vi "UHR-Fleezers Control (host) - 12.6.1.vi"() -> ()   [LabVIEW 2012] (continued)
        w3862 = u32 0 items=["Horizontal", "Vertical", "Central", "1st Diagonal", "2nd Diagonal"] ("Type of Symmetry")
        w3865 = u32 0 items=["Horizontal", "Vertical", "Central", "1st Diagonal", "2nd Diagonal"] ("Type of Symmetry")
        w3894 = u32 0 items=["Horizontal", "Vertical", "Central", "1st Diagonal", "2nd Diagonal"] ("Type of Symmetry")
        n2514 = Unbundle(w3802) -> (w3801:u32[], w3799:u32[], w3797:u32[])
        n2515 = To Double Precision Float(number=w3801) -> (double precision float=w3800:dbl[])
        n2516 = To Double Precision Float(number=w3799) -> (double precision float=w3798:dbl[])
        n2517 = To Double Precision Float(number=w3797) -> (double precision float=w3790:dbl[])
        n2518 = Index Array(array=w3923, index=10) -> (element=w3929:waveform(dbl))
        n2519 = Index Array(array=w3923, index=11) -> (element=w3926:waveform(dbl))
        n2520 = local read "Cycles/step (MCL)"() -> (w3879:u64)
        n2521 = Index Array(array=w3923, index="Channel") -> (element=w3925:waveform(dbl))
        n2522 = Unbundle(w3831) -> ("New Image"=w3830:T2, "New Image"=w3829:T2, "New Image"=w3803:T2, "New Image"=w3804:T2, "New Image"=w3805:T2)
        n2523 = local read "Scan steps (MCL)"() -> (w3792:u64)
        n2524 = Unbundle By Name(w3929) -> ("Y"=w3881:dbl[])
        n2525 = Unbundle By Name(w3926) -> ("Y"=w3883:dbl[])
        n2526 = local read "Scan lines (y)"() -> (w3793:u64)
        n2527 = local read "N APD Samp/step"() -> (w3795:dbl)
        n2528 = Unbundle By Name(w3925) -> ("Y"=w3888:dbl[])
        n2529 = call "downsample 1D array - double.vi"("Ave N"=w3879, "Array In"=w3881) -> ("Array Out"=w3880:dbl[])  [unwired: 1 out]
        n2530 = call "downsample 1D array - double.vi"("Ave N"=w3879, "Array In"=w3883) -> ("Array Out"=w3882:dbl[])  [unwired: 1 out]
        n2531 = call "downsample 1D array - double.vi"("Ave N"=w3879, "Array In"=w3888) -> ("Array Out"=w3887:dbl[])  [unwired: 1 out]
        n2532 = Multiply(x=w3792, y=u64 2) -> (x*y=w3794:u64)
        n2533 = feedback #11(w3798) -> (w3856:dbl[])
        n2534 = Build Array (concatenate)(w3856, w3798) -> (w3855:dbl[])
        n2535 = feedback #12(w3790) -> (w3791:dbl[])
        n2536 = Build Array (concatenate)(w3791, w3790) -> (w3789:dbl[])
        n2537 = Select(t=w3798, s=w3796, f=w3855) -> (s? t:f=w3840:dbl[])
        n2538 = feedback-in #11(w3840) -> ()
        n2539 = Select(t=w3790, s=w3796, f=w3789) -> (s? t:f=w3814:dbl[])
        n2540 = feedback-in #12(w3814) -> ()
        n2541 = feedback #13(w3800) -> (w3949:dbl[])
        n2542 = Build Array (concatenate)(w3949, w3800) -> (w3931:dbl[])
        n2543 = Select(t=w3800, s=w3796, f=w3931) -> (s? t:f=w3935:dbl[])
        n2544 = feedback-in #13(w3935) -> ()
        n2545 = feedback #14(w3880) -> (w3937:dbl[])
        n2546 = Build Array (concatenate)(w3937, w3880) -> (w3928:dbl[])
        n2547 = feedback #15(w3887) -> (w3947:dbl[])
        n2548 = Build Array (concatenate)(w3947, w3887) -> (w3946:dbl[])
        n2549 = feedback #16(w3882) -> (w3939:dbl[])
        n2550 = Build Array (concatenate)(w3939, w3882) -> (w3940:dbl[])
        n2551 = Select(t=w3880, s=w3796, f=w3928) -> (s? t:f=w3884:dbl[])
        n2552 = feedback-in #14(w3884) -> ()
        n2553 = Select(t=w3887, s=w3796, f=w3946) -> (s? t:f=w3886:dbl[])
        n2554 = feedback-in #15(w3886) -> ()
        n2555 = Select(t=w3882, s=w3796, f=w3940) -> (s? t:f=w3885:dbl[])
        n2556 = feedback-in #16(w3885) -> ()
        n2557 = call "integrate 1D array interval - double.vi"("Ave N"=w3795, "Array In"=w3840) -> ("Array Out"=w3851:dbl[])  [unwired: 1 out]
        n2558 = call "integrate 1D array interval - double.vi"("Ave N"=w3795, "Array In"=w3814) -> ("Array Out"=w3825:dbl[])  [unwired: 1 out]
        n2559 = call "integrate 1D array interval - double.vi"("Ave N"=w3795, "Array In"=w3935) -> ("Array Out"=w3934:dbl[])  [unwired: 1 out]
        n2560 = Array Size(array=w3851) -> (size(s)=w3852:i32)
        n2561 = Array Size(array=w3825) -> (size(s)=w3826:i32)
        n2562 = Array Size(array=w3934) -> (size(s)=w3936:i32)
        n2563 = Multiply(x=w3793, y=w3794) -> (x*y=w3854:u64)
        n2564 = Multiply(x=w3793, y=w3794) -> (x*y=w3828:u64)
        n2565 = Multiply(x=w3793, y=w3794) -> (x*y=w3944:u64)
        n2566 = Subtract(x=w3854, y=w3852) -> (x-y=w3845:u64)
        n2567 = call-poly <vilib>:"Mean.vi"("X"=w3851) -> ("mean"=w3842:dbl)  [unwired: 1 out]
        n2568 = Subtract(x=w3828, y=w3826) -> (x-y=w3819:u64)
        n2569 = call-poly <vilib>:"Mean.vi"("X"=w3825) -> ("mean"=w3816:dbl)  [unwired: 1 out]
        n2570 = Subtract(x=w3944, y=w3936) -> (x-y=w3878:u64)
        n2571 = call-poly <vilib>:"Mean.vi"("X"=w3934) -> ("mean"=w3875:dbl)  [unwired: 1 out]
        n2572 = call-poly <vilib>:"Mean.vi"("X"=w3884) -> ("mean"=w3868:dbl)  [unwired: 1 out]
        n2573 = call-poly <vilib>:"Mean.vi"("X"=w3886) -> ("mean"=w3873:dbl)  [unwired: 1 out]
        n2574 = call-poly <vilib>:"Mean.vi"("X"=w3885) -> ("mean"=w3871:dbl)  [unwired: 1 out]
        n2575 = Initialize Array(1.0 ("element"), w3845) -> (w3841:dbl[])
        n2576 = Initialize Array(1.0 ("element"), w3819) -> (w3815:dbl[])
        n2577 = Initialize Array(1.0 ("element"), w3878) -> (w3869:dbl[])
        n2578 = Multiply(x=w3841, y=w3842) -> (x*y=w3843:dbl[])
        n2579 = Multiply(x=w3815, y=w3816) -> (x*y=w3817:dbl[])
        n2580 = Multiply(x=w3869, y=w3875) -> (x*y=w3876:dbl[])
        n2581 = Multiply(x=w3869, y=w3871) -> (x*y=w3872:dbl[])
        n2582 = Multiply(x=w3869, y=w3873) -> (x*y=w3874:dbl[])
        n2583 = Multiply(x=w3869, y=w3868) -> (x*y=w3870:dbl[])
        n2584 = Build Array (concatenate)(w3851, w3843) -> (w3853:dbl[])
        n2585 = Build Array (concatenate)(w3825, w3817) -> (w3827:dbl[])
        n2586 = Build Array (concatenate)(w3934, w3876) -> (w3943:dbl[])
        n2587 = Build Array (concatenate)(w3884, w3870) -> (w3938:dbl[])
        n2588 = Build Array (concatenate)(w3886, w3874) -> (w3942:dbl[])
        n2589 = Build Array (concatenate)(w3885, w3872) -> (w3941:dbl[])
        n2590 = Reshape Array(w3853, w3793, w3794) -> (w3849:dbl[][])
        n2591 = Reshape Array(w3827, w3793, w3794) -> (w3823:dbl[][])
        n2592 = Reshape Array(w3943, w3793, w3794) -> (w3921:dbl[][])
        n2593 = Reshape Array(w3938, w3793, w3794) -> (w3904:dbl[][])
        n2594 = Reshape Array(w3942, w3793, w3794) -> (w3896:dbl[][])
        n2595 = Reshape Array(w3941, w3793, w3794) -> (w3911:dbl[][])
        n2596 = Array Subset(array=w3849, index (col)=0 ("index"), length (col)=w3792) -> (w3848:dbl[][])  [unwired: 2 in]
        n2597 = Array Subset(array=w3849, index (col)=w3792) -> (w3846:dbl[][])  [unwired: 3 in]
        n2598 = Array Subset(array=w3823, index (col)=0 ("index"), length (col)=w3792) -> (w3822:dbl[][])  [unwired: 2 in]
        n2599 = Array Subset(array=w3823, index (col)=w3792) -> (w3820:dbl[][])  [unwired: 3 in]
        n2600 = Array Subset(array=w3911, index (col)=0 ("index"), length (col)=w3792) -> (w3916:dbl[][])  [unwired: 2 in]
        n2601 = Array Subset(array=w3911, index (col)=w3792) -> (w3914:dbl[][])  [unwired: 3 in]
        n2602 = Array Subset(array=w3921, index (col)=0 ("index"), length (col)=w3792) -> (w3920:dbl[][])  [unwired: 2 in]
        n2603 = Array Subset(array=w3921, index (col)=w3792) -> (w3918:dbl[][])  [unwired: 3 in]
        n2604 = Array Subset(array=w3896, index (col)=0 ("index"), length (col)=w3792) -> (w3902:dbl[][])  [unwired: 2 in]
        n2605 = Array Subset(array=w3896, index (col)=w3792) -> (w3900:dbl[][])  [unwired: 3 in]
        n2606 = Array Subset(array=w3904, index (col)=0 ("index"), length (col)=w3792) -> (w3909:dbl[][])  [unwired: 2 in]
        n2607 = Array Subset(array=w3904, index (col)=w3792) -> (w3907:dbl[][])  [unwired: 3 in]
        n2608 = for {
          tunnel: w3848 -> [w3953] mode=indexing
          tunnel: [w3952] -> w3847 mode=indexing
          workers-P: _ -> [_]
          n2609 = Reverse 1D Array(array=w3953) -> (reversed array=w3952:dbl[])
        }
        n2610 = for {
          tunnel: w3822 -> [w3951] mode=indexing
          tunnel: [w3950] -> w3821 mode=indexing
          workers-P: _ -> [_]
          n2611 = Reverse 1D Array(array=w3951) -> (reversed array=w3950:dbl[])
        }
        n2612 = for {
          tunnel: w3916 -> [w3959] mode=indexing
          tunnel: [w3958] -> w3915 mode=indexing
          workers-P: _ -> [_]
          n2613 = Reverse 1D Array(array=w3959) -> (reversed array=w3958:dbl[])
        }
        n2614 = for {
          tunnel: w3920 -> [w3961] mode=indexing
          tunnel: [w3960] -> w3919 mode=indexing
          workers-P: _ -> [_]
          n2615 = Reverse 1D Array(array=w3961) -> (reversed array=w3960:dbl[])
        }
        n2616 = for {
          tunnel: w3902 -> [w3955] mode=indexing
          tunnel: [w3954] -> w3901 mode=indexing
          workers-P: _ -> [_]
          n2617 = Reverse 1D Array(array=w3955) -> (reversed array=w3954:dbl[])
        }
        n2618 = for {
          tunnel: w3909 -> [w3957] mode=indexing
          tunnel: [w3956] -> w3908 mode=indexing
          workers-P: _ -> [_]
          n2619 = Reverse 1D Array(array=w3957) -> (reversed array=w3956:dbl[])
        }
        n2620 = Index Array(array=w3921, index (row)=0) -> (element=→"Waveform Graph":dbl[])  [unwired: 1 in]
        n2621 = Add(x=w3847, y=w3846) -> (x+y=w3833:dbl[][])
        n2622 = Add(x=w3821, y=w3820) -> (x+y=w3807:dbl[][])
        n2623 = Add(x=w3915, y=w3914) -> (x+y=w3913:dbl[][])
        n2624 = Add(x=w3919, y=w3918) -> (x+y=w3893:dbl[][])
        n2625 = Add(x=w3901, y=w3900) -> (x+y=w3899:dbl[][])
        n2626 = Add(x=w3908, y=w3907) -> (x+y=w3906:dbl[][])
        n2627 = Divide(x=w3899, y=2) -> (x/y=w3897:dbl[][])
        n2628 = Divide(x=w3913, y=2) -> (x/y=w3858:dbl[][])
        n2629 = To Single Precision Float(number=w3893) -> (single precision float=w3892:sgl[][])
        n2630 = To Single Precision Float(number=w3833) -> (single precision float=w3837:sgl[][])
        n2631 = To Single Precision Float(number=w3807) -> (single precision float=w3811:sgl[][])
        n2632 = Divide(x=w3906, y=2) -> (x/y=w3860:dbl[][])
        n2633 = Transpose 2D Array(2D array=w3897) -> (transposed array=→"Data map":dbl[][])
        n2634 = To Single Precision Float(number=w3858) -> (single precision float=w3864:sgl[][])
        n2635 = To Single Precision Float(number=w3860) -> (single precision float=w3861:sgl[][])
        n2636 = call "IMAQ ArrayToImage"("Image Pixels (Float)"=w3892, "Image"=w3830) -> ("Image Out"=w3895:T2)  [unwired: 8 in, 1 out]
        n2637 = call "IMAQ ArrayToImage"("Image Pixels (Float)"=w3837, "Image"=w3829) -> ("Image Out"=w3839:T2)  [unwired: 8 in, 1 out]
        n2638 = call "IMAQ ArrayToImage"("Image Pixels (Float)"=w3811, "Image"=w3803) -> ("Image Out"=w3813:T2)  [unwired: 8 in, 1 out]
        n2639 = call "IMAQ ArrayToImage"("Image Pixels (Float)"=w3864, "Image"=w3804) -> ("Image Out"=w3866:T2)  [unwired: 8 in, 1 out]
        n2640 = call "IMAQ Symmetry"("Type of Symmetry"=w3894, "Image Src"=w3895) -> ("Image Dst Out"=w3890:T2)  [unwired: 3 in, 1 out]
        n2641 = call "IMAQ ArrayToImage"("Image Pixels (Float)"=w3861, "Image"=w3805) -> ("Image Out"=w3863:T2)  [unwired: 8 in, 1 out]
        n2642 = call "IMAQ Symmetry"("Type of Symmetry"=w3838, "Image Src"=w3839) -> ("Image Dst Out"=w3835:T2)  [unwired: 3 in, 1 out]
        n2643 = call "IMAQ Symmetry"("Type of Symmetry"=w3812, "Image Src"=w3813) -> ("Image Dst Out"=w3809:T2)  [unwired: 3 in, 1 out]
        n2644 = call "IMAQ Symmetry"("Type of Symmetry"=w3865, "Image Src"=w3866) -> ("Image Dst Out"=→"Detection Laser X":T2)  [unwired: 3 in, 1 out]
        n2645 = call "IMAQ Symmetry"("Type of Symmetry"=w3862, "Image Src"=w3863) -> ("Image Dst Out"=→"Detection Laser Y":T2)  [unwired: 3 in, 1 out]
        n2646 = call "IMAQ Set Simple Calibration"("Calibration Axis Info"=T36 {"Origin Pixel"={"X"=0.0, "Y"=0.0}, "Angle Relative to Horizontal (deg)"=0.0, "Axis Reference"=0}, "Grid Descriptor"=T37 {"X Step"=0.3, "Y Step"=0.3, "Unit"=enum."Undefined"}, "Image"=w3890) -> ("Calibrated Image"=→"APD 1":T2)  [unwired: 7 in, 1 out]
        n2647 = call "IMAQ Set Simple Calibration"("Calibration Axis Info"=T36 {"Origin Pixel"={"X"=0.0, "Y"=0.0}, "Angle Relative to Horizontal (deg)"=0.0, "Axis Reference"=0}, "Grid Descriptor"=T37 {"X Step"=0.3, "Y Step"=0.3, "Unit"=enum."Undefined"}, "Image"=w3835) -> ("Calibrated Image"=→"APD 2":T2)  [unwired: 7 in, 1 out]
        n2648 = call "IMAQ Set Simple Calibration"("Calibration Axis Info"=T36 {"Origin Pixel"={"X"=0.0, "Y"=0.0}, "Angle Relative to Horizontal (deg)"=0.0, "Axis Reference"=0}, "Grid Descriptor"=T37 {"X Step"=0.3, "Y Step"=0.3, "Unit"=enum."Undefined"}, "Image"=w3809) -> ("Calibrated Image"=→"APD 3":T2)  [unwired: 7 in, 1 out]
      }
    }
    n2649 = case "For computing FFTs for display" shown="True" "Compute FFT" {
      tunnel: w3306 -> [_ w4433]
      frame False {
      }
      frame True {
        n2650 = Build Array("FFT 1 Choice 1", "FFT 1 Choice 2", "FFT 2 Choice 1", "FFT 2 Choice 2") -> (w4426:u16[])
        n2651 = Array Size(array=w4433) -> (size(s)=w4432:i32)
        n2652 = feedback-in #17(w4426) -> ()
        n2653 = feedback #17(u16[] [100, 100, 100, 100]) -> (w4427:u16[])
        n2654 = feedback-in #18("# Spectra to Ave.") -> ()
        n2655 = feedback #18("# Spectra to Ave.") -> (w4424:dbl)
        n2656 = Not Equal?(x="# Spectra to Ave.", y=w4424) -> (x != y?=w4423:bool)
        n2657 = Not Equal?(x=w4426, y=w4427) -> (x != y?=w4425:bool)
        n2658 = feedback #19(1.0) -> (w4410:dbl)
        n2659 = Compound Arithmetic op=OR("Reset FFT", w4425, w4423) -> (w4408:bool)
        n2660 = Select(t=1.0, s=w4408, f=w4410) -> (s? t:f=w4412:dbl)
        n2661 = Greater?(x=w4412, y="# Spectra to Ave.") -> (0:w4431:bool)
        n2662 = Increment(x=w4412) -> (x+1=w4411:dbl)
        n2663 = feedback-in #19(w4411) -> ()
        n2664 = local read "DMA Update Period (s)"() -> (w4406:dbl)
        n2665 = Multiply(x="# Spectra to Ave.", y=w4406) -> (x*y=→"Ave. Time (s)":dbl)
        n2666 = Build Array(cluster{"f0":dbl, "df":dbl, "magnitude":dbl[]} {"f0"=0.0, "df"=0.0, "magnitude"=[]} ("PSD")) -> (w4415:cluster{"f0":dbl, "df":dbl, "magnitude":dbl[]}[])
        n2667 = Build Array(w4415, w4415, w4415, w4415) -> (w4417:T46)
        n2668 = feedback #20(w4417) -> (w4422:T46)
        n2669 = for {
          N: 4 -> [_]
          tunnel: w4426 -> [w4455] mode=indexing
          tunnel: w4433 -> [w4456]
          tunnel: w4432 -> [w4458]
          tunnel: w4408 -> [w4451]
          tunnel: w4431 -> [w4450]
          tunnel: "# Spectra to Ave." -> [w4449]
          tunnel: [w4448] -> w4421 mode=indexing
          tunnel: w4422 -> [w4453] mode=indexing
          tunnel: [w4452] -> w4409 mode=indexing
          tunnel: w4412 -> [w4447]
          n2670 = Less?(x=w4455, y=w4458) -> (x < y?=w4457:bool)
          n2671 = Index Array(array=w4456, index=w4455) -> (element=w4454:waveform(dbl))
          n2672 = case shown="True" w4457 {
            tunnel: w4454 -> [_ w4475]
            tunnel: w4453 -> [w4460 w4473]
            tunnel: [w4460 w4461] -> w4452
            tunnel: w4451 -> [_ w4472]
            tunnel: w4450 -> [_ w4465]
            tunnel: w4449 -> [_ w4464]
            tunnel: [cluster{"f0":dbl, "df":dbl, "magnitude":dbl[]} {"f0"=0.0, "df"=0.0, "magnitude"=[]} ("PSD") w4466] -> w4448
            tunnel: w4447 -> [_ w4463]
            frame False {
            }
            frame True {
              n2673 = call <vilib>:"Std Deviation and Variance.vi"("X"=w4475) -> ("mean"=w4476:dbl)  [unwired: 1 in, 2 out]
              n2674 = Subtract(x=w4475, y=w4476) -> (x-y=w4474:waveform(dbl))
              n2675 = xnode "Spectral Measurements"("Signals"=w4474) -> ("PSD"=w4468:cluster{"f0":dbl, "df":dbl, "magnitude":dbl[]})  [unwired: 1 in, 1 out]
              n2676 = case shown="False" w4472 {
                tunnel: w4473 -> [w4485 _]
                tunnel: [w4481 w4490] -> w4461
                tunnel: w4468 -> [w4484 w4491]
                tunnel: w4465 -> [w4483 _]
                frame False {
                  n2677 = Build Array (concatenate)(w4485, w4484) -> (w4482:cluster{"f0":dbl, "df":dbl, "magnitude":dbl[]}[])
                  n2678 = case shown="True" w4483 {
                    tunnel: w4482 -> [w4486 w4489]
                    tunnel: [w4486 w4487] -> w4481
                    frame False {
                    }
                    frame True {
                      n2679 = Delete From Array(array=w4489, index=0) -> (array with subset deleted=w4487:cluster{"f0":dbl, "df":dbl, "magnitude":dbl[]}[])  [unwired: 1 in, 1 out]
                    }
                  }
                }
                frame True {
                  n2680 = Build Array(w4491) -> (w4490:cluster{"f0":dbl, "df":dbl, "magnitude":dbl[]}[])
                }
              }
              n2681 = for {
                tunnel: w4461 -> [w4480] mode=indexing
                tunnel: [w4479] -> w4471 mode=indexing
                workers-P: _ -> [_]
                n2682 = Unbundle By Name(w4480) -> ("magnitude"=w4479:dbl[])
              }
              n2683 = Transpose 2D Array(2D array=w4471) -> (transposed array=w4470:dbl[][])
              n2684 = for {
                tunnel: w4470 -> [w4478] mode=indexing
                tunnel: [w4477] -> w4469 mode=indexing
                workers-P: _ -> [_]
                n2685 = Add Array Elements(numeric array=w4478) -> (sum=w4477:dbl)
              }
              n2686 = Select(t=w4464, s=w4465, f=w4463) -> (s? t:f=w4462:dbl)
              n2687 = Divide(x=w4469, y=w4462) -> (x/y=w4467:dbl[])
              n2688 = Bundle By Name(cluster=w4468, "magnitude"=w4467) -> (w4466:cluster{"f0":dbl, "df":dbl, "magnitude":dbl[]})
            }
          }
        }
        n2689 = case shown="True" w4408 {
          tunnel: w4409 -> [w4440 w4446]
          tunnel: [w4440 w4441] -> w4407
          frame False {
          }
          frame True {
            n2690 = Array Subset(array=w4446, index (row)=0 ("index"), length (row)=4 ("length"), index (col)=0 ("index"), length (col)=1 ("length")) -> (w4441:T46)
          }
        }
        n2691 = feedback-in #20(w4407) -> ()
        n2692 = Split 1D Array(array=w4421, index=2) -> (first subarray=→"FFT 1":cluster{"f0":dbl, "df":dbl, "magnitude":dbl[]}[], second subarray=→"FFT 2":cluster{"f0":dbl, "df":dbl, "magnitude":dbl[]}[])
      }
    }
    n2693 = Index Array(array=w3304, index=4) -> (element=w3360:waveform(dbl))
    n2694 = Index Array(array=w3304, index=7) -> (element=w3357:waveform(dbl))
    n2695 = Divide(x="T1 offset_x (mV)", y=1000.0) -> (x/y=w3361:dbl)
    n2696 = feedback-in #21("Calibration") -> ()
    n2697 = feedback #21(u16 1 ("Calibration")) -> (w3379:u16)
    n2698 = Divide(x="T2 offset_x (mV)", y=1000.0) -> (x/y=w3359:dbl)
    n2699 = case shown="2" "Calibration" {
      tunnel: "T1 alpha_x (nm/V)" -> [_ w3754 w3775]
      tunnel: "T1 kappa_x (pN/nm)" -> [_ _ w3765]
      tunnel: "T2 alpha_x (nm/V)" -> [_ w3753 w3773]
      tunnel: "T2 kappa_x (pN/nm)" -> [_ _ w3766]
      tunnel: w3360 -> [w3736 w3751 w3771]
      tunnel: w3357 -> [w3735 w3749 w3769]
      tunnel: [w3736 w3748 w3768] -> w3388
      tunnel: [w3735 w3747 w3767] -> w3387
      tunnel: ["T1 X (V)" ("Label.Text") "T1 X (nm)" ("Label.Text") "T1 X (pN)" ("Label.Text")] -> w3376
      tunnel: ["T2 X (V)" ("Label.Text") "T2 X (nm)" ("Label.Text") "T2 X (pN)" ("Label.Text")] -> w3375
      tunnel: ["Position (V)" ("Label.Text") "Position (nm)" ("Label.Text") "Force (pN)" ("Label.Text")] -> w3377
      tunnel: w3359 -> [_ w3739 w3758]
      tunnel: w3361 -> [_ w3742 w3760]
      tunnel: ["Mean (V)" ("Label.Text") "Mean (nm)" ("Label.Text") "Mean (pN)" ("Label.Text")] -> w3372
      tunnel: ["Difference (V)" ("Label.Text") "Difference (nm)" ("Label.Text") "Difference (pN)" ("Label.Text")] -> w3312
      frame 0, Default {
      }
      frame 1 {
        n2700 = Unbundle By Name(w3751) -> ("Y"=w3755:dbl[])
        n2701 = Unbundle By Name(w3749) -> ("Y"=w3740:dbl[])
        n2702 = Subtract(x=w3755, y=w3742) -> (x-y=w3743:dbl[])
        n2703 = Subtract(x=w3740, y=w3739) -> (x-y=w3741:dbl[])
        n2704 = Multiply(x=w3741, y=w3753) -> (x*y=w3750:dbl[])
        n2705 = Multiply(x=w3754, y=w3743) -> (x*y=w3752:dbl[])
        n2706 = Bundle By Name(cluster=w3749, "Y"=w3750) -> (w3747:waveform(dbl))
        n2707 = Bundle By Name(cluster=w3751, "Y"=w3752) -> (w3748:waveform(dbl))
      }
      frame 2 {
        n2708 = Unbundle By Name(w3771) -> ("Y"=w3776:dbl[])
        n2709 = Unbundle By Name(w3769) -> ("Y"=w3774:dbl[])
        n2710 = Subtract(x=w3774, y=w3758) -> (x-y=w3759:dbl[])
        n2711 = Subtract(x=w3776, y=w3760) -> (x-y=w3761:dbl[])
        n2712 = Compound Arithmetic op=MULTIPLY(w3759, w3773, w3766) -> (w3770:dbl[])
        n2713 = Compound Arithmetic op=MULTIPLY(w3765, w3775, w3761) -> (w3772:dbl[])
        n2714 = Bundle By Name(cluster=w3769, "Y"=w3770) -> (w3767:waveform(dbl))
        n2715 = Bundle By Name(cluster=w3771, "Y"=w3772) -> (w3768:waveform(dbl))
      }
    }
    n2716 = case shown="True" "Read Lateness and Rel Phase" {
      tunnel: w3178 -> [w3690 w3724]
      tunnel: w3177 -> [w3691 w3723]
      tunnel: [w3690 w3696] -> w3354
      tunnel: [w3691 w3695] -> w3353
      frame False {
      }
      frame True {
        n2717 = xnode "Read/Write Control"("FPGA VI Reference In"=w3724, "error in"=w3723) -> ("FPGA VI Reference Out"=w3698:T20, "error out"=w3697:errorcluster, "GI Relative phase"=→"GI relative phase":i16, "Relative phase"=→"Relative phase (AI1)":i16, "AI Late Counter"=→"Late Counter (AI1)":u8, "GI Late Counter"=→"GI Late Counter":u8, "MCL Late Counter"=→"MCL Late Counter":u8, "MCL Relative Phase"=→"Relative Phase (MCL)":i16, "APD Acq Relative Phase"=→"APD Acq Relative Phase":i16, "APD 1 Gate Relative Phase"=→"APD 1 Gate Relative Phase":i16, "APD 2 Gate Relative Phase"=→"APD 2 Gate Relative Phase":i16, "APD Acq Late Counter"=→"APD Acq Late Counter":u8, "APD 1 Gate Late Counter"=→"APD 1 Gate Late Counter":u8, "APD 2 Gate Late Counter"=→"APD 2 Gate Late Counter":u8, "Green FB Relative Phase"=→"Relative phase (Green FB)":i16, "GI Relative phase 2"=→"GI relative phase 2":i16, "GI Late Counter 2"=→"GI Late Counter 2":u8, "Trap Pos FIFO Timeout"=→"Trap Pos FIFO Timeout":u16, "Trap AI FIFO Timeout"=→"Trap AI FIFO Timeout":u16, "RI Late Counter"=→"RI Late Counter":u8, "RI Relative phase"=→"RI relative phase":i16, "Green Late Counter"=→"Green AI Late Counter":u8, "BI Late Counter (AO)"=→"Late Counter (BI AO)":u8, "Blue Late Counter (D)"=→"Late Counter (BI DO)":u8, "BI Relative phase (AO)"=→"Relative phase (BI AO)":i16, "BI Relative phase (D)"=→"Relative phase (BI DO)":i16, "DIO Relative phase"=→"DIO Relative phase":i16)
        n2718 = xnode "Read/Write Control"("FPGA VI Reference In"=w3698, "error in"=w3697) -> ("FPGA VI Reference Out"=w3696:T20, "error out"=w3695:errorcluster, "APD 3 Gate Late Counter"=→"APD 3 Gate Late Counter":u8, "APD 3 Gate Relative Phase"=→"APD 3 Gate Relative Phase":i16)
      }
    }
    n2719 = Not Equal?(x=w3379, y="Calibration") -> (x != y?=w3338:bool)
    n2720 = case shown="True" w3338 {
      tunnel: w3377 -> [_ w3729]
      tunnel: w3376 -> [_ w3728]
      tunnel: w3375 -> [_ w3727]
      tunnel: w3372 -> [_ w3726]
      tunnel: w3312 -> [_ w3725]
      frame False {
      }
      frame True {
        n2721 = property on="Force" class="WFChart (strict)"("YScale.NameLbl.Text"=w3729) -> ()  [unwired: 2 in, 2 out]
        n2722 = property on="T2 X" class="DigNum (strict)"("Caption.Text"=w3727) -> ()  [unwired: 2 in, 2 out]
        n2723 = property on="T1 X" class="DigNum (strict)"("Caption.Text"=w3728) -> ()  [unwired: 2 in, 2 out]
        n2724 = property on="Mean" class="DigNum (strict)"("Caption.Text"=w3726) -> ()  [unwired: 2 in, 2 out]
        n2725 = property on="Difference" class="DigNum (strict)"("Caption.Text"=w3725) -> ()  [unwired: 2 in, 2 out]
      }
    }
    n2726 = Unbundle By Name(w3360) -> ("Y"=w3363:dbl[])
    n2727 = Unbundle By Name(w3357) -> ("Y"=w3366:dbl[])
    n2728 = Subtract(x=w3363, y=w3361) -> (x-y=w3364:dbl[])
    n2729 = Subtract(x=w3366, y=w3359) -> (x-y=w3365:dbl[])
    n2730 = Multiply(x=w3365, y="T2 alpha_x (nm/V)") -> (x*y=w3160:dbl[])
    n2731 = Multiply(x="T1 alpha_x (nm/V)", y=w3364) -> (x*y=w3161:dbl[])
    n2732 = Not(x="Trap Trig. Fl.") -> (.not. x?=w3197:bool)
    n2733 = Multiply(x=w3387, y=-1.0) -> (x*y=w3368:waveform(dbl))
    n2734 = Subtract(x=w3161, y=w3160) -> (x-y=w3356:dbl[])
    n2735 = Unbundle By Name(w3387) -> ("Y"=w3328:dbl[])
    n2736 = Unbundle By Name(w3388) -> ("Y"=w3162:dbl[])
    n2737 = Negate(x=w3356) -> (-x=w3158:dbl[])
    n2738 = Build Array(w3388, w3368) -> (→"Force":waveform(dbl)[])
    n2739 = Subtract(x=w3158, y="Offset (nm)") -> (x-y=w3326:dbl[])
    n2740 = call-poly <vilib>:"Mean.vi"("X"=w3328) -> ("mean"=w3164:dbl)  [unwired: 1 out]
    "T2 X" <- w3164
    n2741 = Negate(x=w3328) -> (-x=w3329:dbl[])
    n2742 = call-poly <vilib>:"Mean.vi"("X"=w3162) -> ("mean"=w3165:dbl)  [unwired: 1 out]
    "T1 X" <- w3165
    n2743 = Negate(x=w3164) -> (-x=w3163:dbl)
    n2744 = Bundle By Name(cluster=w3360, "Y"=w3326) -> (w3303:waveform(dbl))
    "Bead Separation" <- w3303
    n2745 = Add(x=w3162, y=w3329) -> (x+y=w3330:dbl[])
    n2746 = Add(x=w3165, y=w3163) -> (x+y=w3374:dbl)
    n2747 = Subtract(x=w3165, y=w3163) -> (x-y=→"Difference":dbl)
    n2748 = Divide(x=w3330, y=2.0) -> (x/y=→"Vec Mean of T1 T2":dbl[])
    n2749 = Divide(x=w3374, y=2.0) -> (x/y=w3332:dbl)
    "Mean" <- w3332
    n2750 = feedback-in #22("Trap Trig. Fl.") -> ()
    n2751 = feedback #22("Trap Trig. Fl.") -> (w3195:bool)
    n2752 = And(x=w3197, y=w3195) -> (x .and. y?=w3196:bool)
    n2753 = case "If have just turned off triggering" shown="True" w3196 {
      tunnel: w3178 -> [_ w3525]
      tunnel: w3177 -> [_ w3524]
      frame False {
      }
      frame True {
        w3523 = FALSE ("FPGA Trap Trig")
        n2754 = xnode "Read/Write Control"("FPGA VI Reference In"=w3525, "error in"=w3524, "FPGA Trap Trig"=w3523) -> ("FPGA VI Reference Out"=w3522:T20, "error out"=w3521:errorcluster)
        n2755 = xnode "Read/Write Control"("FPGA VI Reference In"=w3522, "error in"=w3521, "TTrig?"=w3523) -> ()  [unwired: 2 out]
        n2756 = local write "Initializing"(FALSE ("Initializing")) -> ()
        n2757 = local write "Triggered"(FALSE ("Triggered")) -> ()
        n2758 = local write "Waiting"(FALSE ("Waiting")) -> ()
      }
    }
    n2759 = Not(x=w3195) -> (.not. x?=w3208:bool)
    n2760 = And(x="Trap Trig. Fl.", y=w3208) -> (x .and. y?=w3205:bool)
    n2761 = local read "Tether"() -> (w3333:bool)
    n2762 = Or(x=w3205, y="Reinitialize") -> (x .or. y?=w3191:bool)
    n2763 = feedback #23(w3201) -> (w3206:string)
    n2764 = Select(t=w3201, s=w3205, f=w3206) -> (s? t:f=w3200:string)
    n2765 = Select(t=w3201, s="Reinitialize", f=w3200) -> (s? t:f=w3199:string)
    n2766 = feedback #24(0) -> (w3203:i32)
    n2767 = feedback #25(w3326) -> (w3325:dbl[])
    n2768 = Build Array (concatenate)(w3326, w3325) -> (w3159:dbl[])
    n2769 = case "For determining if there is a tether still" shown="True" w3333 {
      tunnel: w3332 -> [_ w3649]
      frame False {
      }
      frame True {
        n2770 = Greater?(x="Lost Tether Alarm Threshold (pN)", y=w3649) -> (0:w3647:bool)
        n2771 = case shown="True" w3647 {
          frame False {
          }
          frame True {
            w3650 = FALSE ("Value (Signaling)")
            n2772 = flat-sequence {
              frame #0 {
                # "stop only if saving"
                n2773 = local read "Saving..."() -> (w3662:bool)
                n2774 = And(x=w3662, y="TA Cancel Save?") -> (x .and. y?=w3661:bool)
                n2775 = local write "Stop Saving"(w3661) -> ()
              }
              frame #1 {
                n2776 = case shown="True" "TA Green Off?" {
                  frame False {
                  }
                  frame True {
                    w3665 = FALSE ("Fl. Triggered...")
                    n2777 = local write "Fl. Triggered..."(w3665) -> ()
                    n2778 = property on="Green Laser ON" class="Bool (strict)"("Val(Sgnl)"=w3665) -> ()  [unwired: 2 in, 2 out]
                  }
                }
              }
            }
            n2779 = local read "Time tether formed"() -> (w3656:timestamp)
            n2780 = Get Date/Time In Seconds() -> (seconds since 1Jan1904=w3657:timestamp)
            n2781 = Subtract(x=w3657, y=w3656) -> (x-y=w3655:dbl)
            n2782 = Number To Decimal String(number=w3655) -> (decimal integer string=w3652:string)  [unwired: 1 out]
            n2783 = local read "Messages"() -> (w3659:string)
            n2784 = call <vilib>:"Beep.vi"() -> ()  [unwired: 3 in, 9 out]
            n2785 = Concatenate Strings("Lost tether (" ("Message to add"), w3652, " s)." ("string")) -> (w3654:string)
            n2786 = local write "Tether"(FALSE ("Tether")) -> ()
            n2787 = call "Update messages.vi"("Message to add"=w3654, "Old message string"=w3659) -> ("New message string"=w3658:string)
            n2788 = local write "Messages"(w3658) -> ()
            n2789 = property on="Fl. Triggered..." class="Bool (strict)"("Val(Sgnl)"=w3650) -> ()  [unwired: 2 in, 2 out]
            n2790 = local write "Dip for Protein"(w3650) -> ()
            n2791 = property on="Trap Pos. FB ON" class="Bool (strict)"("Val(Sgnl)"=w3650) -> ()  [unwired: 2 in, 2 out]
            n2792 = property on="Trap Trig. Fl." class="Bool (strict)"("Val(Sgnl)"=w3650) -> ()  [unwired: 2 in, 2 out]
          }
        }
      }
    }
    n2793 = case "For triggering actions based on the trap position (e.g., turning the excitation laser on if trap under feedback moves so far)" shown="True" "Trap Trig. Fl." {
      tunnel: w3186 -> [_ w3538]
      tunnel: w3199 -> [_ w3537]
      tunnel: ["" ("t") w3536] -> w3207
      tunnel: w3191 -> [_ w3535]
      tunnel: [0 ("t") w3534] -> w3204
      tunnel: w3203 -> [_ w3533]
      tunnel: w3178 -> [_ w3532]
      tunnel: w3177 -> [_ w3531]
      frame False {
      }
      frame True {
        n2794 = case shown="\"Wait for trigger\"" w3537 {
          tunnel: w3538 -> [w3555 _ _ w3603]
          tunnel: [w3552 w3584 "" ("t") w3606] -> w3536
          tunnel: w3535 -> [_ _ _ w3594]
          tunnel: [w3551 w3581 0 ("t") w3595] -> w3534
          tunnel: w3533 -> [_ w3583 _ w3601]
          tunnel: w3532 -> [w3540 w3578 _ w3597]
          tunnel: w3531 -> [w3539 w3577 _ w3596]
          frame "Wait for trigger" {
            n2795 = local read "Trap Trig. (FPGA)"() -> (w3543:bool)
            n2796 = Subtract(x=w3555, y="Mean T1 Position\nto compare (nm)") -> (x-y=w3548:dbl[])
            n2797 = call <vilib>:"Std Deviation and Variance.vi"("X"=w3548) -> ("mean"=→"mean":dbl, "standard deviation"=→"standard\ndeviation":dbl)  [unwired: 1 in, 1 out]
            n2798 = Array Max & Min(array=w3548) -> (max value=→"max value":dbl, min value=→"min value":dbl)  [unwired: 2 out]
            n2799 = Greater?(x=w3548, y="Threshold (nm)") -> (0:w3558:bool[])
            n2800 = case shown="True" w3543 {
              tunnel: w3540 -> [_ w3564]
              tunnel: w3539 -> [_ w3563]
              tunnel: [FALSE ("TTrig?") w3562] -> w3546
              frame False {
              }
              frame True {
                n2801 = xnode "Read/Write Control"("FPGA VI Reference In"=w3564, "error in"=w3563) -> ("TTrig?"=w3562:bool)  [unwired: 2 out]
              }
            }
            n2802 = Or Array Elements(Boolean array=w3558) -> (logical OR=w3545:bool)
            n2803 = Select(t=w3546, s=w3543, f=w3545) -> (s? t:f=w3544:bool)
            n2804 = Not(x=w3543) -> (.not. x?=w3542:bool)
            n2805 = And(x=w3544, y=w3542) -> (x .and. y?=w3541:bool)
            n2806 = Select(t="Triggered", s=w3544, f="Wait for trigger") -> (s? t:f=w3552:string)
            n2807 = case shown="True" w3544 {
              tunnel: [0 0] -> w3551
              tunnel: w3540 -> [_ w3569]
              tunnel: w3539 -> [_ w3568]
              frame False {
                "Waiting" <- TRUE ("Waiting")
              }
              frame True {
                n2808 = xnode "Read/Write Control"("FPGA VI Reference In"=w3569, "error in"=w3568, "TTrig?"=FALSE) -> ()  [unwired: 2 out]
                n2809 = local read "Messages"() -> (w3572:string)
                n2810 = call <vilib>:"Beep.vi"() -> ()  [unwired: 12 in]
                n2811 = call "Update messages.vi"("Message to add"="Unwinding trigger.", "Old message string"=w3572) -> ("New message string"=w3573:string)
                n2812 = local write "Messages"(w3573) -> ()
                n2813 = local write "Waiting"(FALSE ("Waiting")) -> ()
                "Triggered" <- TRUE ("Triggered")
              }
            }
            n2814 = case "Only need to turn on laser if host triggered" shown="True" w3541 {
              frame False {
              }
              frame True {
                n2815 = property on="Green Laser ON" class="Bool (strict)"("Val(Sgnl)"=TRUE ("Value (Signaling)")) -> ()  [unwired: 2 in, 2 out]
              }
            }
          }
          frame "Triggered" {
            n2816 = local read "Trap Trig. (FPGA)"() -> (w3580:bool)
            n2817 = Increment(x=w3583) -> (x+1=w3581:i32)
            n2818 = Greater Or Equal?(x=w3581, y="Fl. ON time (n)") -> (x >= y?=w3579:bool)
            n2819 = Select(t="Wait for trigger", s=w3579, f="Triggered" ("t")) -> (s? t:f=w3584:string)
            n2820 = And(x=w3579, y=w3580) -> (x .and. y?=w3576:bool)
            n2821 = case shown="True" w3576 {
              tunnel: w3578 -> [_ w3588]
              tunnel: w3577 -> [_ w3587]
              frame False {
              }
              frame True {
                n2822 = xnode "Read/Write Control"("FPGA VI Reference In"=w3588, "error in"=w3587, "FPGA Trap Trig"=TRUE) -> ()  [unwired: 2 out]
              }
            }
            n2823 = case shown="True" w3579 {
              frame False {
              }
              frame True {
                w3590 = FALSE ("Value (Signaling)")
                n2824 = local write "Triggered"(w3590) -> ()
                n2825 = local write "Waiting"(TRUE ("Waiting")) -> ()
                n2826 = property on="Green Laser ON" class="Bool (strict)"("Val(Sgnl)"=w3590) -> ()  [unwired: 2 in, 2 out]
              }
            }
          }
          frame "Do nothing" {
          }
          frame "Initialize", Default {
            n2827 = Increment(x=w3601) -> (x+1=w3605:i32)
            n2828 = Select(t=1, s=w3594, f=w3605) -> (s? t:f=w3595:i32)
            n2829 = feedback #26(w3603) -> (w3609:dbl[])
            n2830 = Build Array (concatenate)(w3603, w3609) -> (w3602:dbl[])
            n2831 = Greater Or Equal?(x=w3595, y="Wait to get offset (n)") -> (x >= y?=w3598:bool)
            n2832 = Select(t=w3603, s=w3594, f=w3602) -> (s? t:f=w3604:dbl[])
            n2833 = feedback-in #26(w3604) -> ()
            n2834 = call-poly <vilib>:"Mean.vi"("X"=w3604) -> ("mean"=w3599:dbl)  [unwired: 1 out]
            n2835 = local write "Mean T1 Position\nto compare (nm)"(w3599) -> ()
            n2836 = case shown="True" w3594 {
              tunnel: w3597 -> [_ w3615]
              tunnel: w3596 -> [_ w3614]
              frame False {
              }
              frame True {
                w3611 = FALSE ("FPGA Trap Trig")
                n2837 = xnode "Read/Write Control"("FPGA VI Reference In"=w3615, "error in"=w3614, "FPGA Trap Trig"=w3611) -> ("FPGA VI Reference Out"=w3613:T20, "error out"=w3612:errorcluster)
                n2838 = xnode "Read/Write Control"("FPGA VI Reference In"=w3613, "error in"=w3612, "TTrig?"=w3611) -> ()  [unwired: 2 out]
              }
            }
            n2839 = Select(t="Wait for trigger", s=w3598, f="Initialize") -> (s? t:f=w3606:string)
            n2840 = case shown="True" w3598 {
              tunnel: w3599 -> [_ w3618]
              tunnel: w3597 -> [_ w3627]
              tunnel: w3596 -> [_ w3626]
              frame False {
                n2841 = local write "Waiting"(FALSE ("Waiting")) -> ()
                "Initializing" <- TRUE ("Initializing")
              }
              frame True {
                n2842 = local read "Threshold (nm)"() -> (w3630:dbl)
                n2843 = local read "AOM X Cal (nm/MHz)"() -> (w3629:dbl)
                n2844 = Add(x=w3618, y=w3630) -> (x+y=w3631:dbl)
                n2845 = Divide(x=w3631, y=w3629) -> (x/y=w3628:dbl)
                n2846 = call "IR AOM freq to word.vi"("Frequency In (MHz)"=w3628) -> ("Frequency Word Out (double)"=w3625:dbl)
                n2847 = local write "Initializing"(FALSE ("Initializing")) -> ()
                n2848 = local write "Waiting"(TRUE ("Waiting")) -> ()
                n2849 = To Quad Integer(1:w3625) -> (0:w3624:i64)
                n2850 = xnode "Read/Write Control"("FPGA VI Reference In"=w3627, "error in"=w3626, "FPGA TTrig Thresh"=w3624) -> ("FPGA VI Reference Out"=w3621:T20, "error out"=w3620:errorcluster)
                n2851 = xnode "Read/Write Control"("FPGA VI Reference In"=w3621, "error in"=w3620, "FPGA Trap Trig"=TRUE) -> ()  [unwired: 2 out]
              }
            }
          }
        }
      }
    }
    n2852 = feedback-in #23(w3207) -> ()
    n2853 = feedback-in #24(w3204) -> ()
    n2854 = Split 1D Array(array=w3159, index=w3221) -> (first subarray=w3322:dbl[])  [unwired: 1 out]
    n2855 = feedback-in #25(w3322) -> ()
    n2856 = call-poly <vilib>:"Mean.vi"("X"=w3322) -> ("mean"=w3321:dbl)  [unwired: 1 out]
    "Bead Mean (nm)" <- w3321
    n2857 = Subtract(x=w3322, y=w3321) -> (x-y=w3320:dbl[])
    n2858 = Square(x=w3320) -> (x^2=w3319:dbl[])
    n2859 = call-poly <vilib>:"Mean.vi"("X"=w3319) -> ("mean"=w3318:dbl)  [unwired: 1 out]
    n2860 = Square Root(x=w3318) -> (sqrt(x)=w3317:dbl)
    n2861 = Multiply(x=10.0, y=w3317) -> (x*y=→"RMS (Ang)":dbl)
    n2862 = xnode ("Read/Write Control")("FPGA VI Reference In"=w3354, "error in"=w3353) -> ("FPGA VI Reference Out"=w3189:T20, "error out"=w3188:errorcluster, "AI2 Y Sum Set 1"=w3452:i16, "AI2 Y Sum Set 2"=w3451:i16, "AI1 X Set 1"=w3253:fxp<+/-,16,1>, "AI1 X Set 2"=w3252:fxp<+/-,16,1>, "Trap Pos FB Int Signal"=→"Trap Pos FB Int Signal":fxp<+/-,24,9>, "Trap Pos FB Int-Norm Signal"=→"Trap Pos FB Int-Norm Signal":fxp<+/-,16,1>, "Trap Pos FB Action"=w3246:i64, "Scanning"=→"AOD Scanning":bool, "Scan I"=→"AOD Scan I":u64, "Scanning MCL"=w3454:bool, "Scan I (MCL)"=→"MCL Scan I":u64, "Green FB Sum"=w3391:i16, "Trap Pos FB Action"=w3176:i64, "TTrig Fin Thresh"=w3172:i64, "Red FB Intensity"=w3153:i16, "Blue Intensity"=w3148:i16)
    "MCL Scanning" <- w3454
    "Trap Pos FB Action" <- w3246
    n2863 = Divide(x=w3153, y=3276.7) -> (x/y=w3152:dbl)
    "Red laser intensity (V)" <- w3152
    n2864 = Divide(x=w3148, y=3276.7) -> (x/y=w3147:dbl)
    "Blue laser intensity (V)" <- w3147
    n2865 = Divide(x=w3391, y=3276.7) -> (x/y=w3151:dbl)
    "Green laser intensity (V)" <- w3151
    n2866 = local read "FB Trig Integrate"() -> (w3170:u32)
    n2867 = Divide(x=w3176, y=w3170) -> (x/y=w3169:dbl)
    "TTrig Sig (Int)" <- w3169
    n2868 = Bundle(w3151, w3152, w3147) -> (→"Fluorescence laser intensities plot":cluster{dbl, dbl, dbl})  [unwired: 1 in]
    n2869 = Divide(x=w3172, y=w3170) -> (x/y=w3167:dbl)
    "TTrig Fin Thresh (Int)" <- w3167
    n2870 = local read "AOM X Cal (nm/MHz)"() -> (w3175:dbl)
    n2871 = local read "AI2 (V)"() -> (w3453:cluster{"Set 1":dbl, "Set 2":dbl})
    n2872 = Bundle By Name(cluster=w3453, "Set 1"=w3452, "Set 2"=w3451) -> (w3449:cluster{"Set 1":dbl, "Set 2":dbl})
    n2873 = Divide(x=w3246, y=327.67) -> (x/y=→"Action (%)":dbl)
    n2874 = local read "Trap X (AI1)"() -> (w3266:T10)
    n2875 = call "IR AOM word double to freq.vi"("Frequency Word In (double)"=w3167) -> ("Frequency Out (MHz)"=w3166:dbl)
    n2876 = call "IR AOM word double to freq.vi"("Frequency Word In (double)"=w3169) -> ("Frequency Out (MHz)"=w3168:dbl)
    n2877 = Divide(x=w3449, y=3276.7) -> (x/y=w3448:cluster{"Set 1":dbl, "Set 2":dbl})
    n2878 = Multiply(x=w3168, y=w3175) -> (x*y=w3174:dbl)
    "TTrig Sig (nm)" <- w3174
    n2879 = Multiply(x=w3166, y=w3175) -> (x*y=w3173:dbl)
    "TTrig Fin Thresh (nm)" <- w3173
    n2880 = local write "AI2 (V)"(w3448) -> ()
    n2881 = Bundle(cluster=w3266, "Trap 1"=w3253, "Trap 2"=w3252) -> (→"Trap X (AI1)":T10)
    n2882 = Bundle(w3174, w3173) -> (→"TTrig":cluster{dbl, dbl})  [unwired: 1 in]
    n2883 = flat-sequence "To save data" {
      tunnel: [w4539] -> w3472
      tunnel: [w4540] -> w3471
      tunnel: w3422 -> [w4533]
      tunnel: w3194 -> [w4537]
      tunnel: ["Save Calibration"] -> w3445
      tunnel: w3442 -> [w4536]
      tunnel: [w4529] -> w3441
      tunnel: [w4526] -> w3440
      tunnel: [w4523] -> w3439
      tunnel: w3421 -> [w4525]
      tunnel: w3336 -> [w4519]
      tunnel: [w4519] -> w3335
      tunnel: ["Start Saving"] -> w3305
      tunnel: [w4513] -> w3234
      tunnel: [w4512] -> w3233
      tunnel: w3472 -> [w4787]
      tunnel: w3471 -> [w4786]
      tunnel: w3235 -> [w4785]
      tunnel: w3445 -> [w4784]
      tunnel: w3441 -> [w4782]
      tunnel: w3440 -> [w4781]
      tunnel: w3439 -> [w4780]
      tunnel: w3314 -> [w4779]
      tunnel: w3346 -> [w4778]
      tunnel: w3335 -> [w4777]
      tunnel: w3305 -> [w4776]
      tunnel: w3303 -> [w4775]
      tunnel: w3133 -> [w4774]
      tunnel: w3234 -> [w4773]
      tunnel: w3233 -> [w4772]
      tunnel: w3232 -> [w4771]
      tunnel: w3155 -> [w4770]
      frame #0 {
        n2884 = Or(x="Save N Sets", y="Start Saving") -> (x .or. y?=w4520:bool)
        n2885 = To Double Precision Float(number=w4536) -> (double precision float=w4530:dbl)
        n2886 = Build Array(w4520, "Save Calibration", w4533, w4525) -> (w4535:bool[])
        n2887 = Compound Arithmetic op=OR("Save Calibration", w4533, w4520, w4525) -> (w4538:bool)
        n2888 = Boolean Array To Number(Boolean array=w4535) -> (number=w4532:u32)
        n2889 = feedback #27(FALSE ("Save APD Data\nwith Trap Data")) -> (w4514:bool)
        n2890 = feedback #28(refnum<k0> refnum) -> (w4541:refnum<file>)
        n2891 = feedback #29(refnum<k0> refnum) -> (w4516:refnum<file>)
        n2892 = feedback #30(FALSE ("Save APD Data\nwith Trap Data")) -> (w4524:bool)
        n2893 = feedback #31(refnum<k0> refnum) -> (w4527:refnum<file>)
        n2894 = feedback #32(0) -> (w4543:i32)
        n2895 = feedback #33() -> (w4531:u32)  [unwired: 1 out]
        n2896 = case shown="True" w4538 {
          tunnel: [w4550 1] -> w4539
          tunnel: w4543 -> [w4552 _]
          tunnel: [w4551 w4583] -> w4540
          tunnel: w4541 -> [w4551 _]
          tunnel: w4537 -> [_ w4601]
          tunnel: w4530 -> [_ w4599]
          tunnel: w4532 -> [_ w4602]
          tunnel: [w4549 w4582] -> w4529
          tunnel: w4531 -> [w4549 _]
          tunnel: [w4548 w4580] -> w4526
          tunnel: w4527 -> [w4548 _]
          tunnel: [w4547 w4579] -> w4523
          tunnel: w4524 -> [w4547 _]
          tunnel: "Start Saving" -> [_ w4577]
          tunnel: w4519 -> [_ w4576]
          tunnel: [w4546 w4568] -> w4512
          tunnel: w4516 -> [w4546 _]
          tunnel: [w4545 w4567] -> w4513
          tunnel: w4514 -> [w4545 _]
          frame False {
            n2897 = Increment(x=w4552) -> (x+1=w4550:i32)
          }
          frame True {
            w4573 = FALSE ("Start Saving")
            w4578 = 9.0  # File Version
            w4585 = FALSE ("prepend array or string size? (T)")
            w4584 = T28."big-endian, network order" ("byte order (0:big-endian, network order)")
            n2898 = local read "BD 1 Frequency 1 (MHz)"() -> (w4598:dbl)
            n2899 = local read "BD 2 Frequency 1 (MHz)"() -> (w4597:dbl)
            n2900 = local read "BD 1 Frequency 2 (MHz)"() -> (w4596:dbl)
            n2901 = local read "BD 2 Frequency 2 (MHz)"() -> (w4595:dbl)
            n2902 = local read "BD 1 Frequency 3 (MHz)"() -> (w4594:dbl)
            n2903 = local read "BD 2 Frequency 3 (MHz)"() -> (w4593:dbl)
            n2904 = Array Size(array=w4576) -> (size(s)=w4575:i32)
            n2905 = To Double Precision Float(number=w4575) -> (double precision float=w4574:dbl)
            n2906 = local write "Save Calibration"(w4573) -> ()
            n2907 = local write "Start Saving"(w4573) -> ()
            n2908 = Build Array("Save APD Data\nwith Trap Data", "Save Trap Pos. Data") -> (w4570:bool[])
            n2909 = Boolean Array To Number(Boolean array=w4570) -> (number=w4569:u32)
            n2910 = Build Array(w4598, w4597, w4596, w4595, w4594, w4593) -> (w4592:dbl[])
            n2911 = case shown="1, Default" w4602 {
              tunnel: w4601 -> [w4674 w4694 w4710 w4748]
              tunnel: w4574 -> [w4679 w4701 w4730 w4767]
              tunnel: w4599 -> [w4678 w4700 w4729 w4766]
              tunnel: [w4675 w4696 w4721 w4758] -> w4590
              tunnel: [w4666 "Cal sets to save" w4711 w4749] -> w4582
              tunnel: w4592 -> [w4676 w4697 w4723 w4760]
              tunnel: "Save APD Data\nwith Trap Data" -> [w4673 _ w4707 w4746]
              tunnel: [w4673 w4688 w4707 w4746] -> w4579
              tunnel: w4578 -> [w4669 w4689 w4705 w4744]
              tunnel: w4577 -> [w4668 _ _ _]
              tunnel: [w4659 w4688 w4704 w4734] -> w4567
              tunnel: "Save Trap Pos. Data" -> [w4659 _ w4704 w4734]
              tunnel: w4569 -> [w4658 _ w4703 w4733]
              frame 1, Default {
                # "timeseries"
                n2912 = case shown="True" "Profile" {
                  tunnel: [w4682 w4686] -> w4663
                  tunnel: [w4682 w4685] -> w4662
                  tunnel: [w4682 w4684] -> w4661
                  tunnel: [w4682 w4683] -> w4660
                  frame False {
                    w4682 = 0.0 ("f")
                  }
                  frame True {
                    n2913 = local read "Current Position"() -> (w4687:cluster{dbl, dbl, dbl})
                    n2914 = local read "Y change (mm)"() -> (w4683:dbl)
                    n2915 = Unbundle(w4687) -> (w4686:dbl, w4685:dbl, w4684:dbl)
                  }
                }
                n2916 = local read "Save ave N"() -> (w4681:dbl)
                n2917 = Multiply(x=w4681, y=w4674) -> (x*y=w4680:dbl)
                n2918 = To Double Precision Float(number=w4658) -> (double precision float=w4672:dbl)
                n2919 = Build Array(w4669, w4674, w4680, w4679, w4678, 0.0 ("f")) -> (w4677:dbl[])
                n2920 = Build Array(w4672, w4663, w4662, w4661, w4660) -> (w4670:dbl[])
                n2921 = Select(t=u32 4000000000, s=w4668, f="N sets to save") -> (s? t:f=w4666:u32)
                n2922 = Build Array (concatenate)(w4677, w4676, w4670) -> (w4675:dbl[])
              }
              frame 2 {
                w4691 = 0.0 ("f")
                w4688 = FALSE ("Save APD Data\nwith Trap Data")
                # "calibration"
                n2923 = Boolean To (0,1)(Boolean=w4688) -> (0, 1=w4693:i16)
                n2924 = To Double Precision Float(number=w4693) -> (double precision float=w4692:dbl)
                n2925 = Build Array(w4692, w4691, w4691, w4691, w4691) -> (w4690:dbl[])
                n2926 = Build Array(w4689, w4694, w4694, w4701, w4700, 1.0 ("t")) -> (w4698:dbl[])
                n2927 = Build Array (concatenate)(w4698, w4697, w4690) -> (w4696:dbl[])
                "Calibrating Trap..." <- TRUE ("Calibrating...")
              }
              frame 4 {
                w4708 = 0.0 ("f")
                # "scan dir (x/y = 0/1)"
                # "cycles/step"
                # "n scans (f/b)"
                # "steps"
                # "freq. range"
                # "AOD raster scan"
                n2928 = local read "Number of F/B Scans (AOD)"() -> (w4715:u16)
                n2929 = local read "Cycles/step (AOD)"() -> (w4717:u64)
                n2930 = local read "Scan Range (MHz)"() -> (w4720:dbl)
                n2931 = local read "Scan steps (AOD)"() -> (w4719:u64)
                n2932 = local read "Scan BD"() -> (w4727:bool)
                n2933 = local read "Save ave N"() -> (w4732:dbl)
                n2934 = Boolean To (0,1)(Boolean=w4727) -> (0, 1=w4726:i16)
                n2935 = To Double Precision Float(number=w4715) -> (double precision float=w4714:dbl)
                n2936 = To Double Precision Float(number=w4719) -> (double precision float=w4718:dbl)
                n2937 = To Double Precision Float(number=w4717) -> (double precision float=w4716:dbl)
                n2938 = To Double Precision Float(number=w4726) -> (double precision float=w4725:dbl)
                n2939 = Multiply(x=w4732, y=w4710) -> (x*y=w4731:dbl)
                n2940 = To Double Precision Float(number=w4703) -> (double precision float=w4709:dbl)
                n2941 = Build Array(w4709, w4708, w4708, w4708, w4708) -> (w4706:dbl[])
                n2942 = local read "N sets should be saved"() -> (w4712:dbl)
                n2943 = Build Array(w4725, w4720, w4718, w4716, w4714) -> (w4722:dbl[])
                n2944 = Build Array(w4705, w4710, w4731, w4730, w4729, 2.0 ("t")) -> (w4724:dbl[])
                n2945 = Round Toward +Infinity(x=w4712) -> (ceil(x): smallest int >= x=w4713:dbl)
                n2946 = Build Array (concatenate)(w4724, w4723, w4706, w4722) -> (w4721:dbl[])
                n2947 = To Unsigned Long Integer(number=w4713) -> (unsigned 32bit integer=w4711:u32)
              }
              frame 8 {
                w4741 = 0.0 ("f")
                # "MCL raster scan"
                n2948 = local read "Number of scans (MCL)"() -> (w4736:u64)
                n2949 = local read "Scan lines (y)"() -> (w4735:u64)
                n2950 = local read "2D or 1D Scan"() -> (w4738:bool)
                n2951 = local read "Scan Range (V)\n(of steps)"() -> (w4757:dbl)
                n2952 = local read "Fast Scan Dir"() -> (w4764:bool)
                n2953 = local read "Cycles/step (MCL)"() -> (w4754:u64)
                n2954 = local read "Scan steps (MCL)"() -> (w4756:u64)
                n2955 = Select(t=w4735, s=w4738, f=w4736) -> (s? t:f=w4737:u64)
                n2956 = Boolean To (0,1)(Boolean=w4738) -> (0, 1=w4740:i16)
                n2957 = local read "Save ave N"() -> (w4769:dbl)
                n2958 = local read "Initial X"() -> (w4743:dbl)
                n2959 = local read "Initial Y"() -> (w4742:dbl)
                n2960 = To Double Precision Float(number=w4740) -> (double precision float=w4739:dbl)
                n2961 = Boolean To (0,1)(Boolean=w4764) -> (0, 1=w4763:i16)
                n2962 = To Double Precision Float(number=w4737) -> (double precision float=w4752:dbl)
                n2963 = To Double Precision Float(number=w4756) -> (double precision float=w4755:dbl)
                n2964 = To Double Precision Float(number=w4754) -> (double precision float=w4753:dbl)
                n2965 = To Double Precision Float(number=w4763) -> (double precision float=w4762:dbl)
                n2966 = Multiply(x=w4769, y=w4748) -> (x*y=w4768:dbl)
                n2967 = To Double Precision Float(number=w4733) -> (double precision float=w4747:dbl)
                n2968 = local read "N sets should be saved (MCL)"() -> (w4750:dbl)
                n2969 = Build Array(w4747, w4739, w4741, w4741, w4741) -> (w4745:dbl[])
                n2970 = Build Array(w4762, w4757, w4755, w4753, w4752, w4743, w4742) -> (w4759:dbl[])
                n2971 = Build Array(w4744, w4748, w4768, w4767, w4766, 3.0 ("t")) -> (w4761:dbl[])
                n2972 = Round Toward +Infinity(x=w4750) -> (ceil(x): smallest int >= x=w4751:dbl)
                n2973 = Build Array (concatenate)(w4761, w4760, w4745, w4759) -> (w4758:dbl[])
                n2974 = To Unsigned Long Integer(number=w4751) -> (unsigned 32bit integer=w4749:u32)
              }
            }
            n2975 = local read "Index"() -> (w4607:dbl)
            n2976 = call "Create new save file.vi"("Insert"="", "Ext"=".dat", "Index In"=w4607) -> ("Path Out"=w4563:path, "Index Out"=w4581:dbl)
            n2977 = local write "Save file name"(w4563) -> ()
            n2978 = local write "Index"(w4581) -> ()
            n2979 = local write "Save index"(w4581) -> ()
            n2980 = Array Size(array=w4590) -> (size(s)=w4591:i32)
            n2981 = Open/Create/Replace File(file path (use dialog)=w4563, operation (0:open)=T29."create", access (0:read/write)=enum16{"read/write", "read-only", "write-only"}."write-only") -> (refnum out=w4604:refnum<file>)  [unwired: 1 in, 4 out]
            n2982 = local write "Saving..."(TRUE ("Saving...")) -> ()
            n2983 = To Double Precision Float(number=w4591) -> (double precision float=w4589:dbl)
            n2984 = String Length(string="Comment (data description)") -> (length=w4588:i32)
            n2985 = To Double Precision Float(number=w4588) -> (double precision float=w4587:dbl)
            n2986 = Deny Access(7:w4604) -> (3:w4603:refnum<file>)  [unwired: 1 in, 2 out]